vi "UHR-Fleezers Control (host) - 10.7.vi"() -> ()   [LabVIEW 2010] (continued)
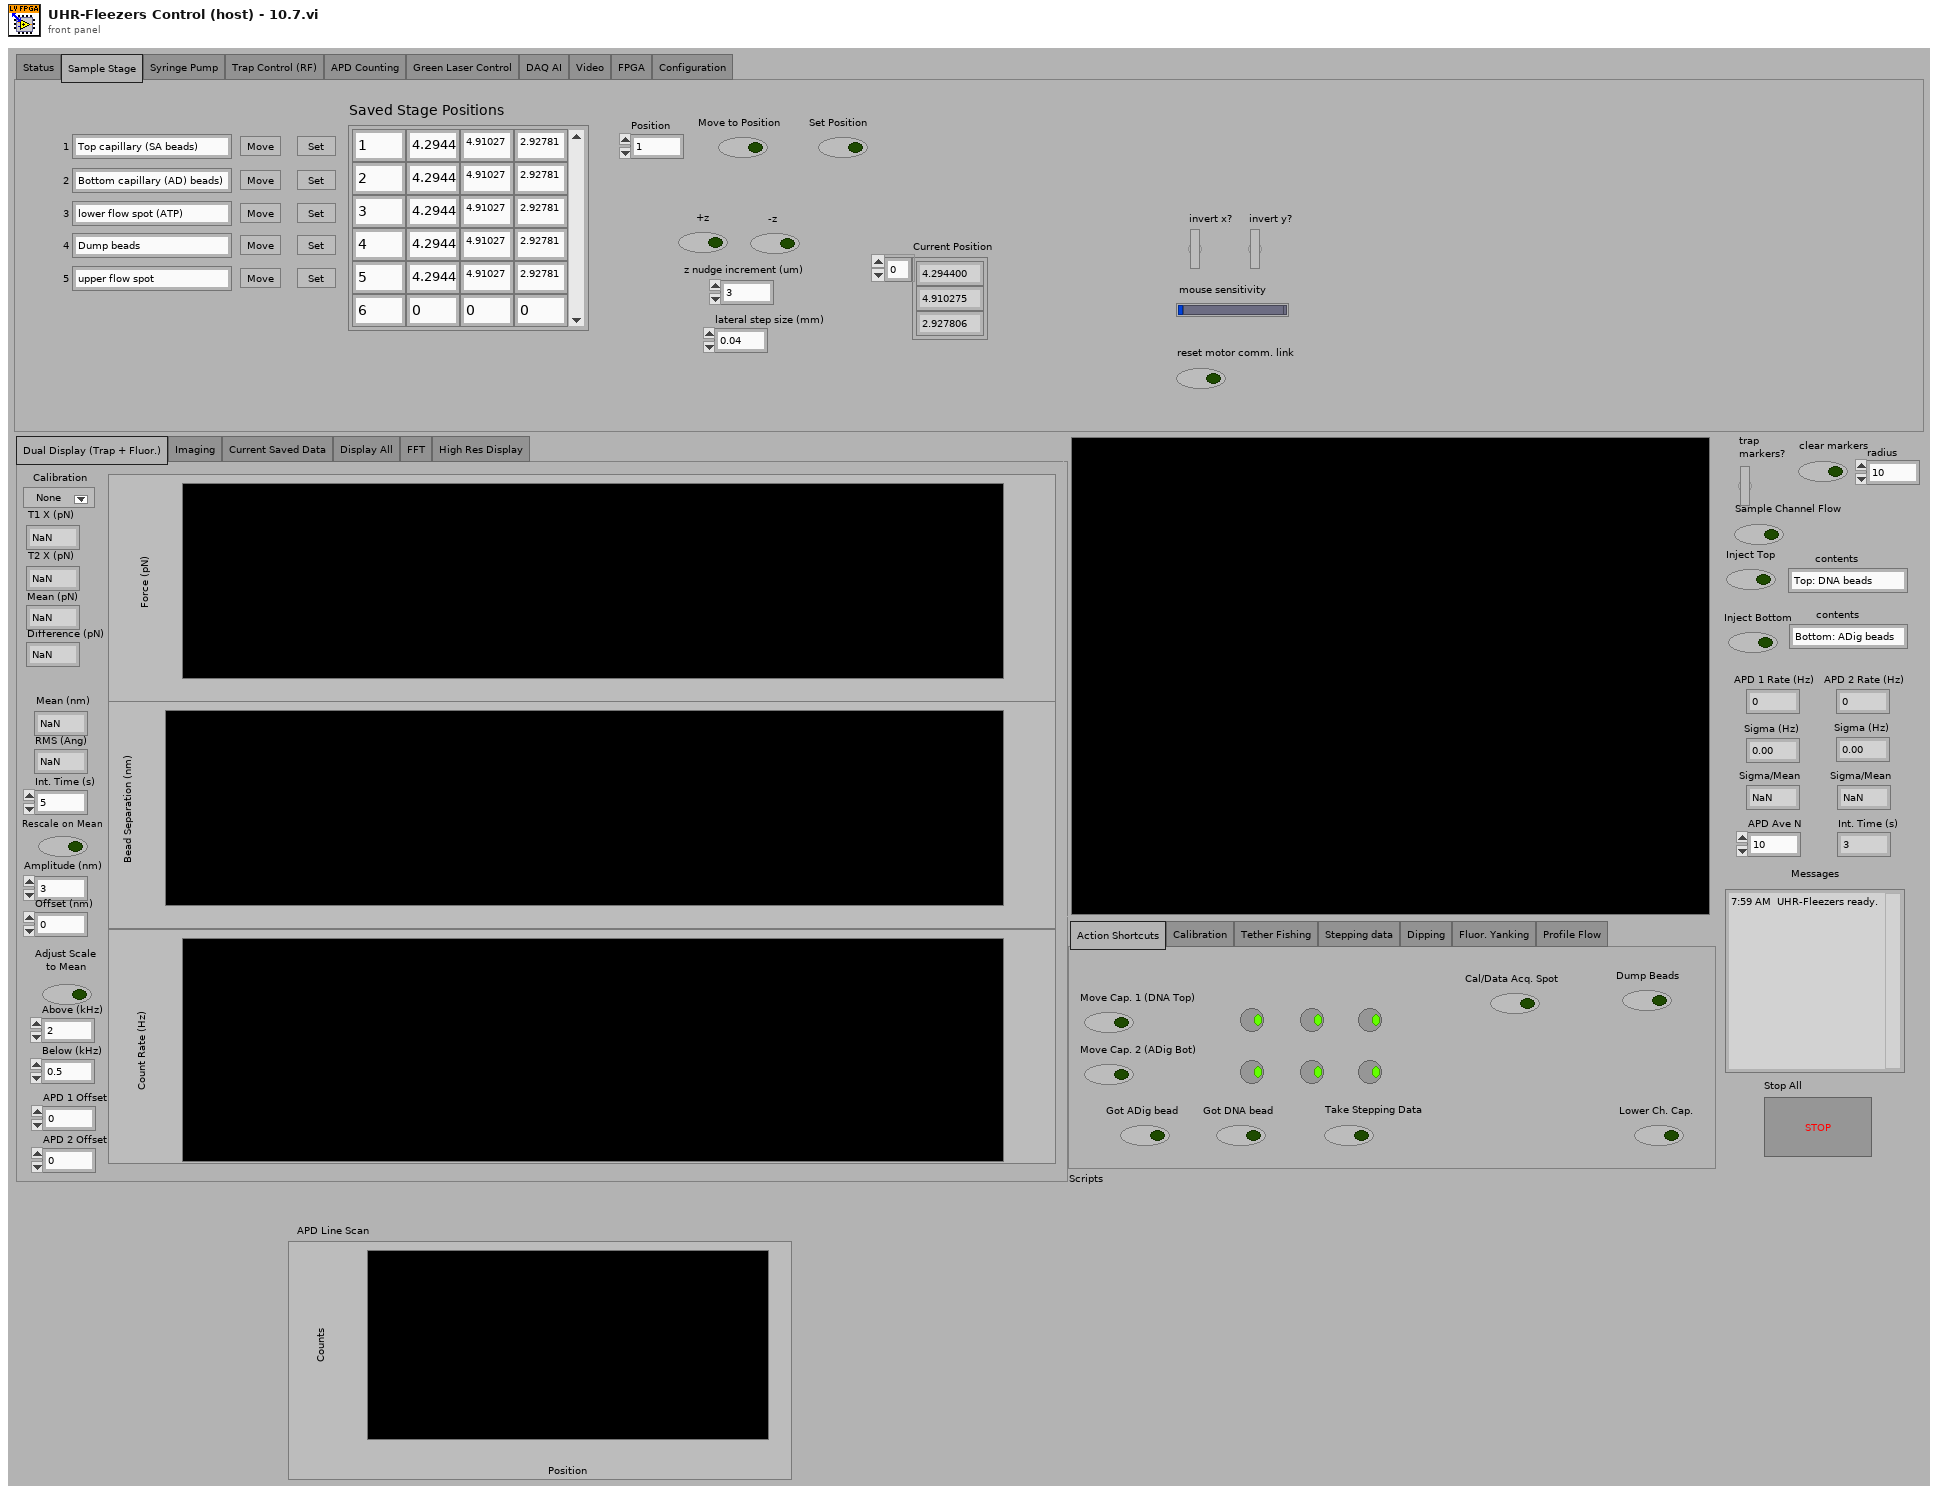
[diagram p1: front panel]
types:
  T1 = enum32{"Action Shortcuts", "Calibration", "Tether Fishing", "Stepping data", "Dipping", "Fluor. Yanking", "Profile Flow"}
  T2 = typedef "IMAQ Image.ctl" = refnum<image>
  T3 = enum32{"Dual Display (Trap + Fluor.)", "Imaging", "Current Saved Data", "Display All", "FFT", "High Res Display"}
  T4 = enum32{"Status", "Sample Stage", "Syringe Pump", "Trap Control (RF)", "APD Counting", "Green Laser Control", "DAQ AI", "Video", "FPGA", "Configuration"}
  T5 = cluster{"Pump 1":cluster{"Diameter (mm)":dbl, "Units":dbl, "Volume":dbl, "Rate":dbl}, "Pump 2":cluster{"Diameter (mm)":dbl, "Units":dbl, "Volume":dbl, "Rate":dbl}, "Pump 3":cluster{"Diameter (mm)":dbl, "Units":dbl, "Volume":dbl, "Rate":dbl}}
  T6 = enum32{"IR Laser Interlacing (Direct RF Board Control Method)", "AOD Raster Scan", "Feedback on Trap Intensity", "Feedback on Trap Position"}
  T7 = typedef "LVPoint32TypeDef.ctl" = cluster{"Horizontal":i32, "Vertical":i32}
  T8 = cluster{"Scan Range AOD (nm) 2":dbl, "Step Size AOD (nm) 2":dbl, "Scan Speed AOD (nm/s) 2":dbl, "Number of scans (AOD) 2":u16, "Label":string}[]
  T9 = cluster{"Set 1":cluster{"proportional gain (Kc)":i16, "integral gain (Kc*Ts/Ti)":i16, "derivative gain (Kc*Td/Ts)":i16}, "Set 2":cluster{"proportional gain (Kc)":i16, "integral gain (Kc*Ts/Ti)":i16, "derivative gain (Kc*Td/Ts)":i16}}
  T10 = cluster{"Trap 1":fxp<+/-,16,1>, "Trap 2":fxp<+/-,16,1>}
  T11 = cluster{"proportional gain (Kc)":fxp<+/-,16,8>, "integral gain (Kc*Ts/Ti)":fxp<+/-,16,8>, "derivative gain (Kc*Td/Ts)":fxp<+/-,16,8>}
  T12 = cluster{"output high":fxp<+/-,16,1>, "output low":fxp<+/-,16,1>}
  T13 = cluster{"Set 1":fxp<+/-,16,1>, "Set 2":fxp<+/-,16,1>}
  T14 = cluster{"proportional gain (Kc)":i16, "integral gain (Kc*Ts/Ti)":i16, "derivative gain (Kc*Td/Ts)":i16}
  T15 = cluster{"Set 1":bool, "Set 2":bool, "Set 3":bool}
  T16 = typedef "LVMinMaxIncTypeDef.ctl" = cluster{"Minimum":dbl, "Maximum":dbl, "Increment":dbl}
  T17 = typedef "Image Type" = u32
  T18 = typedef "nirio_resource_hc.ctl" = tag
  T19 = typedef "openfpgaref.8.6.ctl" = refnum<k20>
  T20 = typedef "niFpgaNodeNameForErrorReporting.ctl" = enum16{"Open FPGA VI Reference", "Read/Write Control", "Invoke Method: Abort", "Invoke Method: Acknowledge IRQ", "Invoke Method: Download", "Invoke Method: FIFO.Configure", "Invoke Method: FIFO.Read", "Invoke Method: FIFO.Start", "Invoke Method: FIFO.Stop", "Invoke Method: FIFO.Write", "Invoke Method: Reset", "Invoke Method: Run", "Invoke Method: Wait on IRQ", "Close FPGA VI Reference"}
  T21 = typedef "niLvFpgaWhatHappensToTopLevelVI.ctl" = enum16{"top level VI scripted behind XNode", "top level VI inlined behind XNode"}
  T22 = enum16{"GET STATUS", "ABS MOVE", "GET POS", "REL MOVE", "INIT", "CLOSE", "HOME", "READ ASCII", "ASCII", "SET ULIM", "STOP", "SET LLIM"}
  T23 = enum16{"CONNECT", "INITIALIZE VALVES", "DISCONNECT", "MOVE VALVE"}
  T24 = cluster{"New Image":T2, "New Image":T2, "New Image":T2, "New Image":T2}
  T25 = enum16{"open", "replace", "create", "open or create", "replace or create", "replace or create with confirmation"}
  T26 = typedef "XDNodeRunTimeDep.lvlib/timing_clust.ctl" = cluster{"Expected End [f-1]":u64, "Actual End [f-1]":u64, "Finished Late? [f-1]":bool, "Expected End [i-1]":u64, "Actual End [i-1]":u64, "Finished Late? [i-1]":bool, "Expected Start [i]":u64, "Actual Start [i]":u64, "Expected Start [f]":u64, "Actual Start [f]":u64, "Source Name":string, "Structure Name":string, "Period":i64, "Deadline":i64, "Offset":i64, "Start":i64, "Priority":i32, "Timeout":i32, "Mode":T27, "Wakeup Reason":T28, "Error":errorcluster, "Source Type":string, "Secondary Source Type":string, "Global End Time":u64, "Global Start Time":u64, "Frame Duration":u64, "Iteration Duration":u64, "Assigned CPU":i32, "I/O Scan Engine Mode":u32}
  T27 = typedef "XDNodeRunTimeDep.lvlib/nitl_modes.ctl" = enum32{"No Change", "Process missed periods, maintain original phase", "Discard missed periods, maintain original phase", "Process missed periods, ignore original phase", "Discard missed periods, ignore original phase"}
  T28 = typedef "XDNodeRunTimeDep.lvlib/wakeup.ctl" = enum32{"Normal", "Aborted", "Asynchronous wakeup", "Timing source error", "Timed loop error", "Timeout"}
  T29 = cluster{"[0]":i32, "[1]":i32, "[2]":i32, "[3]":i32}
  T30 = cluster{"[0]":i32, "[1]":i32, "[2]":i32, "[3]":i32}[]
  T31 = cluster{"Horizontal":i32, "Vertical":i32, "Scrolling":i32}
  T32 = enum32{"Normal Display", "Dual Display (APD)", "FFT", "High Res Display"}
  T33 = cluster{"Origin Pixel":cluster{"X":sgl, "Y":sgl}, "Angle Relative to Horizontal (deg)":sgl, "Axis Reference":u32}
  T34 = typedef "Simple Grid Descriptor" = cluster{"X Step":sgl, "Y Step":sgl, "Unit":T35}
  T35 = typedef "Image Unit" = enum32{"Undefined", "Angström", "Micrometer", "Millimeter", "Centimeter", "Meter", "Kilometer", "Microinch", "Inch", "Feet", "Nautical miles", "Standard miles", "Steps"}
  T36 = cluster{"averaging mode":u16, "weighting mode":u16, "number of averages":u32}
  T37 = cluster{"dB On (F)":bool, "unwrap phase (F)":bool, "convert to degree (F)":bool}
  T38 = cluster{"Green FB Ch 0":i16, "Green FB Ch 1":i16, "Green FB Ch 2":i16}
  T39 = enum16{"big-endian, network order", "native, host order", "little-endian"}
  T40 = cluster{string, string, string, string, string, string, string, string}
  T41 = cluster{string, string, string, string, string, string, string, string, string, string, string, string}
  T42 = cluster{string, string, string, string, string, string, string, string, string, string, string, string, string}
  T43 = cluster{string, string, string, string, string, string, string, string, string, string, string, string, string, string}
  T44 = cluster{"BD 1 Frequency 1 (MHz)":dbl, "BD 1 Frequency 2 (MHz)":dbl}
  T45 = cluster{"f0":dbl, "df":dbl, "magnitude":dbl[]}[][]
  T46 = cluster{"Green FB Ch 0":dbl, "Green FB Ch 1":dbl, "Green FB Ch 2":dbl}
  T47 = enum16{"Always On", "Always Off", "Off While Running"}
  T48 = cluster{"Scan Range AOD (nm) 2":dbl, "Step Size AOD (nm) 2":dbl, "Scan Speed AOD (nm/s) 2":dbl, "Number of scans (AOD) 2":u16, "Label":string}
  T49 = typedef "eventvkey.ctl" = enum16{"ASCII", "Enter", "Return", "Shift", "Ctrl", "Alt", "Cmd", "Opt", "Caps", "NumLock", "Clear", "Break", "Up", "Down", "Left", "Right", "Insert", "Delete", "Home", "End", "PageUp", "PageDown", "Escape", "Help", "Pause", "ScrollLock", "F1", "F2", "F3", "F4", "F5", "F6", "F7", "F8", "F9", "F10", "F11", "F12", "F13", "F14", "F15", "F16", "F17", "F18", "F19", "F20", "F21", "F22", "F23", "F24", "Play", "VolumeUp", "VolumeDown", "Mute", "Two Byte Char"}
  T50 = cluster{"[0]":dbl, "[1]":dbl, "[2]":dbl, "[3]":dbl, "[4]":dbl, "[5]":dbl}
  T51 = cluster{"Diameter (mm)":dbl, "Units":dbl, "Volume":dbl, "Rate":dbl}
  T52 = cluster{"Left":i32, "Top":i32, "Width":u32, "Height":u32}
  T53 = cluster{cluster{"Left":i32, "Top":i32, "Width":u32, "Height":u32}}[]
diagram:
  w63 = T17 2 items=["Grayscale (U8)", "Grayscale (I16)", "Grayscale (SGL)", "Complex (CSG)", "RGB (U32)", "HSL (U32)", "RGB (U64)", "Grayscale (U16)"] ("Image Type")
  w120 = cluster{"output high":i16, "output low":i16} {"output high"=3000, "output low"=0} ("FB output range 1")
  w195 = 10.0 ("y")
  w194 = 32767.0 ("y")
  w210 = 6.0  # clock mult.
  w211 = 49152000.0  # TCXO frequ.
  n1 = Build Array("DIO count 1 (ticks)", "DIO count 2 (ticks)", "DIO count 3 (ticks)") -> (w109:u32[])
  n2 = Multiply(x="APD Integration Time (s)", y=40000000.0) -> (x*y=w127:dbl)
  n3 = Reciprocal(x="APD Integration Time (s)") -> (1/x=w124:dbl)
  n4 = local write "APD Acq Rate (Hz)"(w124) -> ()
  n5 = local read "AO1"() -> (w189:dbl)
  n6 = local read "AO2"() -> (w188:dbl)
  n7 = To Unsigned Long Integer(number=w127) -> (unsigned 32bit integer=w126:u32)
  "APD Int. Count" <- w126
  n8 = local read "Scan Increment (MHz)"() -> (w206:dbl)
  n9 = local read "Continuous MCL Scanning"() -> (w176:bool)
  n10 = local read "Fast Scan Dir"() -> (w175:bool)
  n11 = local read "Trap Intensity\nSetpoints (V)"() -> (w225:cluster{"Set 1":dbl, "Set 2":dbl})
  n12 = local read "Number of scans (MCL)"() -> (w177:u64)
  n13 = Multiply(x=w189, y=w194) -> (x*y=w191:dbl)
  n14 = Multiply(x=w188, y=w194) -> (x*y=w193:dbl)
  n15 = Divide(x=w191, y=w195) -> (x/y=w190:dbl)
  n16 = Divide(x=w193, y=w195) -> (x/y=w192:dbl)
  n17 = To Word Integer(number=w190) -> (16bit integer=w187:i16)
  n18 = To Word Integer(number=w192) -> (16bit integer=w186:i16)
  n19 = Not(x=w175) -> (.not. x?=w170:bool)
  n20 = local read "Cycles/step (MCL)"() -> (w178:u64)
  n21 = Multiply(x=w206, y=1000.0) -> (x*y=w213:dbl)
  n22 = local read "Scan steps (MCL)"() -> (w179:u64)
  n23 = local write "Trap Pos FIFO Timeout"(u16 0 ("Trap Pos FIFO Timeout")) -> ()
  n24 = local read "Desired Scan Incr (V)"() -> (w181:dbl)
  n25 = Scale By Power Of 2(n=48, x=w213) -> (x*2^n=w214:dbl)
  n26 = Multiply(x=w211, y=w210) -> (x*y=w209:dbl)
  n27 = Divide(x=w214, y=w209) -> (x/y=w208:dbl)
  n28 = local read "Number Interlace Sets"() -> (w102:u8)
  n29 = Split 1D Array(array=w109, index=w102) -> (first subarray=w111:u32[])  [unwired: 1 out]
  n30 = Add Array Elements(numeric array=w111) -> (sum=w110:u32)
  n31 = property on="AI Count (ticks)" class="DigNum (strict)"("Val(Sgnl)"="AI Count (ticks)") -> ()  [unwired: 2 in, 2 out]
  n32 = local read "# Samples/channel"() -> (w198:u32)
  n33 = local read "Number of F/B Scans (AOD)"() -> (w199:u16)
  n34 = To Quad Integer(1:w208) -> (0:w205:i64)
  n35 = local read "Not-Interlacing Set"() -> (w101:enum32{"Set 1", "Set 2", "Set 3"})
  n36 = To Unsigned Byte Integer(number=w101) -> (unsigned 8bit integer=w107:u8)
  n37 = Index Array(array=w109, index=w107) -> (element=w108:u32)
  n38 = local read "Feedback On/Off"() -> (w228:cluster{"Set 1":bool, "Set 2":bool})
  n39 = local read "PID Gains"() -> (w220:T9)
  n40 = Divide(x=40000000.0, y="AI Count (ticks)") -> (x/y=w167:dbl)
  n41 = Multiply(x=w181, y=32767.0) -> (x*y=w183:dbl)
  n42 = local read "Scan steps (AOD)"() -> (w204:u64)
  n43 = local read "All FB On/Off"() -> (w229:bool)
  n44 = local read "Cycles/step (AOD)"() -> (w203:u64)
  n45 = local write "AI rate (Hz)"(w167) -> ()
  n46 = Divide(x=w183, y=10.0) -> (x/y=w182:dbl)
  n47 = Multiply(x=w204, y=w203) -> (x*y=w202:u64)
  n48 = Multiply(x=3276.7, y=w225) -> (x*y=w224:cluster{"Set 1":dbl, "Set 2":dbl})
  n49 = To Word Integer(number=w182) -> (16bit integer=w180:i16)
  n50 = Multiply(x=w202, y=u64 2) -> (x*y=w200:u64)
  n51 = local read "Sets to FIFO (Traps)"() -> (w232:T15)
  n52 = Divide(x=w167, y="FPGA Ave.") -> (x/y=w168:dbl)
  n53 = To Word Integer(number=w224) -> (16bit integer=w223:cluster{"Set 1":i16, "Set 2":i16})
  n54 = xnode "Open FPGA VI Reference"("resource name"=T18 "750kHzDAQ") -> ("FPGA VI Reference Out"=w217:T19)  [unwired: 1 in, 1 out]
  n55 = Unbundle By Name(w220) -> ("Set 1"=w219:T14, "Set 2"=w218:T14)
  n56 = Multiply(x=w200, y=w199) -> (x*y=w197:u64)
  n57 = local write "Ave. Rate (Hz)"(w168) -> ()
  n58 = Divide(x=w197, y=w198) -> (x/y=w196:dbl)
  n59 = Unbundle By Name(w223) -> ("Set 1"=w222:i16, "Set 2"=w221:i16)
  n60 = local read "2D or 1D Scan"() -> (w121:bool)
  n61 = local write "Data points/scans"(w197) -> ()
  n62 = local read "Scan BD"() -> (w215:bool)
  n63 = And(x=w228, y=w229) -> (x .and. y?=w227:cluster{"Set 1":bool, "Set 2":bool})
  n64 = local write "Data points/scan (f/b)"(w200) -> ()
  n65 = Reciprocal(x=w168) -> (1/x=w169:dbl)
  n66 = local read "N Acq Sets (Traps + Fl.)"() -> (w160:i16)
  n67 = local write "N sets should be saved"(w196) -> ()
  n68 = Unbundle By Name(w227) -> ("Set 1"=w231:bool, "Set 2"=w230:bool)
  n69 = local read "Interlace"() -> (w103:bool)
  n70 = Select(t=w110, s=w103, f=w108) -> (s? t:f=w100:u32)
  n71 = local write "Update Count (MCL)"(w100) -> ()
  n72 = local write "Total Counts (ticks)"(w100) -> ()
  n73 = xnode "Invoke Method"("FPGA VI Reference In"=w217) -> ("FPGA VI Reference Out"=w119:T19, "error out"=w138:errorcluster)  [unwired: 1 in]
  n74 = local write "Ave. Period (s)"(w169) -> ()
  n75 = property on="2D or 1D Scan" class="Bool (strict)"("Val(Sgnl)"=w121) -> ()  [unwired: 2 in, 2 out]
  n76 = xnode "Read/Write Control"("FPGA VI Reference In"=w118, "error in"=w138, "ai count"="AI Count (ticks)", "Interlace ON/OFF"=w103, "Number Interlace Cycles"=w102, "AI1 Sets to FIFO"=w232, "FB On/Off Set 1"=w231, "FB On/Off Set 2"=w230, "Interlace Off Parameters"=w101, "FB Setpoint Set 1"=w222, "FB Setpoint Set 2"=w221, "FB Gains Set 1"=w219, "FB Gains Set 2"=w218, "FB output range 1"=w120, "FB output range 2"=w120, "Cycles per step"=w203, "Scan BD"=w215, "Number of scans"=w199, "Scan steps"=w204, "Scan freq.  increment"=w205, "AO1"=w187, "AO2"=w186, "Scan freq.  increment (MCL)"=w180, "Scan steps (MCL)"=w179, "Cycles per step (MCL)"=w178, "Number of scans (MCL)"=w177, "MCL count"=w100, "Cont. Scan (MCL)"=w176, "MCL Scan Axis"=w170, "1D or 2D Scan?"=w121, "N of AI1 Int Acq Sets"=w160, "Freq or Amp switch first"="Freq or Amp switch first", "Freq switch delay"="Freq switch delay", "Amp switch delay"="Amp switch delay", "Swap F1 and F2"="Swap F1 and F2", "APD Acq Rate Count"=w126, "APD to FIFO"=FALSE, "APD Gate Operating Mode"="APD Gate", "APD Gate ON Count"="APD Gate ON Count", "APD Gate OFF Count"="APD Gate OFF Count", "Invert APD Gate"="Invert APD Gate", "DIO count 1 (ticks)"="DIO count 1 (ticks)", "DIO count 2 (ticks)"="DIO count 2 (ticks)", "DIO count 3 (ticks)"="DIO count 3 (ticks)", "APD 1 AO scale factor"="APD 1 AO Mult.", "APD 2 AO scale factor"="APD 2 AO Mult.") -> ("FPGA VI Reference Out"=w95:T19, "error out"=w97:errorcluster)  [unwired: 1 in]
  n77 = local read "Green Laser ON/Interlacing"() -> (w98:bool)
  n78 = local read "Green laser mode"() -> (w99:enum32{"Laser ON", "Laser OFF", "Interlace"})
  n79 = local read "GI Frequency, OFF count"() -> (w91:u32)
  n80 = local read "GI Frequency, ON count"() -> (w90:u32)
  n81 = Multiply(x="Current When FB OFF (%)", y=655.35) -> (x*y=w81:dbl)
  n82 = local read "Green FB Count"() -> (w89:u32)
  n83 = Multiply(x="Green FB Setpoint (mV)", y=3.2767) -> (x*y=w78:dbl)
  n84 = To Unsigned Word Integer(number=w81) -> (unsigned 16bit integer=w79:u16)
  n85 = local read "Invert GI"() -> (w93:bool)
  n86 = To Word Integer(number=w78) -> (16bit integer=w76:i16)
  n87 = case shown="True" w98 {
    tunnel: w99 -> [_ w252]
    tunnel: [enum32{"Laser ON", "Laser OFF", "Interlace"}."Laser OFF" ("Green laser mode") w252] -> w92
    frame False {
    }
    frame True {
    }
  }
  n88 = local read "Trap Pos. AI1 X Pre-scale"() -> (w47:u16)
  n89 = local read "Trap Pos FB Monitor\nT1 or T2"() -> (w54:bool)
  n90 = local read "Trap Pos FB Int Count"() -> (w42:u16)
  n91 = local read "Trap Pos FB Negate Action"() -> (w53:bool)
  n92 = local read "Trap Pos. FB Offset Factor"() -> (w52:i64)
  n93 = local read "Trap Pos. FB Mult Factor"() -> (w51:i64)
  n94 = local read "Trap Pos. FB Gains"() -> (w49:T11)
  n95 = local read "Trap Pos. FB Range"() -> (w50:T12)
  n96 = xnode "Read/Write Control"("FPGA VI Reference In"=w95, "error in"=w97, "Green interlace ON count 2"=w90, "Green interlace OFF count 2"=w91, "Invert GI 2"=w93, "Operating Mode 2"=w92, "Green FB Gains"="Green FB Gains", "Green FB Setpoint"=w76, "Green FB On/Off"="Green FB On/Off", "Current Out"=w79, "Green int current ON count adj"="Green int current ON count adj", "Green FB Count"=w89, "Operating Mode"=w92, "Green interlace OFF count"=w91, "Green interlace ON count"=w90, "Invert GI"=w93, "Trap Pos FB Monitor T1 or T2"=w54, "Trap Pos FB Negate Action"=w53, "Trap Pos. FB Offset Factor"=w52, "Trap Pos. FB Mult Factor"=w51, "Trap Pos. FB Range"=w50, "Trap Pos. FB Gains"=w49, "Force feedback"=FALSE, "AI1 X Scale"=w47, "Trap Pos to FIFO"=TRUE, "Trap Pos FB Int Count"=w42) -> ("FPGA VI Reference Out"=w94:T19, "error out"=w96:errorcluster)
  n97 = xnode "Invoke Method"("FPGA VI Reference In"=w94, "error in"=w96, "Depth"="Trap AI FIFO Depth") -> ("FPGA VI Reference Out"=w57:T19, "error out"=w56:errorcluster)
  n98 = xnode "Invoke Method"("FPGA VI Reference In"=w57, "error in"=w56, "Depth"="Trap Position FIFO Depth") -> ("FPGA VI Reference Out"=w44:T19, "error out"=w43:errorcluster)
  n99 = flat-sequence {
    tunnel: w119 -> [w257]
    tunnel: [w257] -> w118
    tunnel: [w256] -> w117
    tunnel: [w255] -> w116
    tunnel: [w253] -> w114
    tunnel: [w254] -> w115
    frame #0 {
      w254 = T16 {"Minimum"=50.0, "Maximum"=100.0, "Increment"=1.0} ("Min Max Inc")
      w253 = T16 {"Minimum"=0.0, "Maximum"=75.0, "Increment"=1.0} ("Data Entry Limits")
      w256 = T16 {"Minimum"=50.0, "Maximum"=100.0, "Increment"=1.0} ("Min Max Inc")
      w255 = T16 {"Minimum"=0.0, "Maximum"=75.0, "Increment"=1.0} ("Data Entry Limits")
      n100 = property on="BD 2 Frequency 1 (MHz)" class="DigNum (strict)"("Data Range"=w254) -> ()  [unwired: 2 in, 2 out]
      n101 = property on="BD 2 Frequency 3 (MHz)" class="DigNum (strict)"("Data Range"=w254) -> ()  [unwired: 2 in, 2 out]
      n102 = property on="BD 2 Frequency 2 (MHz)" class="DigNum (strict)"("Data Range"=w254) -> ()  [unwired: 2 in, 2 out]
      n103 = property on="BD 1 Frequency 1 (MHz)" class="DigNum (strict)"("Data Range"=w256) -> ()  [unwired: 2 in, 2 out]
      n104 = property on="BD 1 Frequency 2 (MHz)" class="DigNum (strict)"("Data Range"=w256) -> ()  [unwired: 2 in, 2 out]
      n105 = property on="BD 1 Frequency 3 (MHz)" class="DigNum (strict)"("Data Range"=w256) -> ()  [unwired: 2 in, 2 out]
      n106 = property on="BD 2 Amplitude 1 (%)" class="DigNum (strict)"("Data Range"=w253) -> ()  [unwired: 2 in, 2 out]
      n107 = property on="BD 2 Amplitude 2 (%)" class="DigNum (strict)"("Data Range"=w253) -> ()  [unwired: 2 in, 2 out]
      n108 = property on="BD 2 Amplitude 3 (%)" class="DigNum (strict)"("Data Range"=w253) -> ()  [unwired: 2 in, 2 out]
      n109 = property on="BD 1 Amplitude 3 (%)" class="DigNum (strict)"("Data Range"=w255) -> ()  [unwired: 2 in, 2 out]
      n110 = property on="BD 1 Amplitude 2 (%)" class="DigNum (strict)"("Data Range"=w255) -> ()  [unwired: 2 in, 2 out]
      n111 = property on="BD 1 Amplitude 1 (%)" class="DigNum (strict)"("Data Range"=w255) -> ()  [unwired: 2 in, 2 out]
      "X RF Frequency Limits (MHz)" <- w256
      "X RF Amplitude Limits (%)" <- w255
      "Y RF Amplitude Limits (%)" <- w253
      "Y RF Frequency Limits (MHz)" <- w254
    }
  }
  n112 = xnode "Invoke Method"("FPGA VI Reference In"=w44, "error in"=w43) -> ("FPGA VI Reference Out"=w14:T19, "error out"=w13:errorcluster)  [unwired: 1 out]
  n113 = flat-sequence "Initial FPGA Loop Relative Phase Adjustment" {
    tunnel: "Initial Phase Adjustment (APD 2 Gate)" -> [w259]
    tunnel: "Initial Phase Adjustment (GI) 2" -> [w260]
    tunnel: "Initial Phase Adj. (MCL)" -> [w261]
    tunnel: w13 -> [w262]
    tunnel: w14 -> [w263]
    tunnel: "Initial Phase Adjustment (GI)" -> [w264]
    tunnel: "Initial Phase Adjustment (AI1)" -> [w265]
    tunnel: [w265] -> w28
    tunnel: [w264] -> w27
    tunnel: [w263] -> w26
    tunnel: [w262] -> w25
    tunnel: [w261] -> w24
    tunnel: [w260] -> w23
    tunnel: [w259] -> w22
    tunnel: [w277] -> w144
    tunnel: [w271] -> w142
    tunnel: "Initial Phase Adjustment (APD Acq)" -> [w270]
    tunnel: "Initial Phase Adjustment (APD 1 Gate)" -> [w269]
    tunnel: "Initial Phase Adjustment (Green FB)" -> [w268]
    tunnel: w28 -> [w276]
    tunnel: w27 -> [w275]
    tunnel: w26 -> [w274]
    tunnel: w25 -> [w273]
    tunnel: w24 -> [w272]
    tunnel: w23 -> [w267]
    tunnel: w22 -> [w266]
    tunnel: w144 -> [w456]
    tunnel: [w457] -> w143
    tunnel: w142 -> [w457]
    tunnel: [w456] -> w141
    tunnel: w143 -> [w460]
    tunnel: w141 -> [w459]
    tunnel: [w462] -> w140
    tunnel: [w461] -> w139
    tunnel: [w649] -> w12
    tunnel: [w650] -> w15
    tunnel: w140 -> [w650]
    tunnel: w139 -> [w649]
    frame #0 {
      n114 = Wait (ms)(milliseconds to wait=u32 1000) -> ()  [unwired: 1 out]
    }
    frame #1 {
      n115 = xnode "Read/Write Control"("FPGA VI Reference In"=w274, "error in"=w273, "Phase count adjustment"=w276, "Phase count adjustment (GI)"=w275, "Phase count adjustment (MCL)"=w272, "Phase Count Adjustment (APD Acq)"=w270, "Phase count adjustment (APD 1 Gate)"=w269, "Phase count adjustment (APD 2 Gate)"=w266, "Phase count adjustment (Green FB)"=w268, "Phase count adjustment (GI) 2"=w267) -> ("FPGA VI Reference Out"=w271:T19, "error out"=w277:errorcluster)
    }
    frame #2 {
      n116 = Wait (ms)(milliseconds to wait=u32 1000) -> ()  [unwired: 1 out]
    }
    frame #3 {
      w458 = TRUE
      n117 = xnode "Read/Write Control"("FPGA VI Reference In"=w460, "error in"=w459, "+ phase"=w458, "+ phase (GI)"=w458, "+ phase (MCL)"=w458, "+ phase (APD Acq)"=w458, "+ phase (APD 1 Gate)"=w458, "+ phase (APD 2 Gate)"=w458, "+ phase (Green FB)"=w458, "+ phase (GI) 2"=w458) -> ("FPGA VI Reference Out"=w461:T19, "error out"=w462:errorcluster)
    }
    frame #4 {
      n118 = Wait (ms)(milliseconds to wait=u32 1000) -> ()  [unwired: 1 out]
    }
  }
  n119 = local read "Phase adj. (Green FB)"() -> (w112:i16)
  n120 = local read "Phase adj. (GI) 2"() -> (w82:i16)
  n121 = local read "Phase adjust (MCL)"() -> (w171:i16)
  n122 = local read "Phase adj. (AI1)"() -> (w173:i16)
  n123 = local read "Phase adj. (GI)"() -> (w172:i16)
  n124 = xnode "Read/Write Control"("FPGA VI Reference In"=w12, "error in"=w15, "Phase count adjustment"=w173, "Phase count adjustment (GI)"=w172, "Phase count adjustment (MCL)"=w171, "Phase Count Adjustment (APD Acq)"="Phase Adj. (APD Acq)", "Phase count adjustment (APD 1 Gate)"="Phase Adj. (APD 1 Gate)", "Phase count adjustment (APD 2 Gate)"="Phase Adj. (APD 2 Gate)", "Phase count adjustment (Green FB)"=w112, "Phase count adjustment (GI) 2"=w82) -> ("FPGA VI Reference Out"=w11:T19, "error out"=w10:errorcluster)
  n125 = call "Initialize RF boards - interlace 3.vi"("error in"=w10, "FPGA VI Reference In"=w11) -> ("FPGA VI Reference Out"=w149:T19)  [unwired: 1 out]
  n126 = call "set RF board frequency - interlace.vi"("Board 2 Frequency Limits"=w115, "Board 1 Frequency Limits"=w117, "FPGA VI Reference In"=w149, "Board 2 Frequency 3 (MHz)"="BD 2 Frequency 3 (MHz)", "Board 1 Frequency 3 (MHz)"="BD 1 Frequency 3 (MHz)", "Board 2 Frequency 2 (MHz)"="BD 2 Frequency 2 (MHz)", "Board 2 Frequency 1 (MHz)"="BD 2 Frequency 1 (MHz)", "Board 1 Frequency 2 (MHz)"="BD 1 Frequency 2 (MHz)", "Board 1 Frequency 1  (MHz)"="BD 1 Frequency 1 (MHz)") -> ("error out"=w243:errorcluster, "FPGA VI Reference Out"=w244:T19)  [unwired: 1 in]
  n127 = call "set RF board amplitude - interlace.vi"("Board 2 Amplitude Limits"=w114, "Board 1 Amplitude Limits"=w116, "error in"=w243, "FPGA VI Reference In"=w244, "Board 2 Amplitude 3 (%)"="BD 2 Amplitude 3 (%)", "Board 1 Amplitude 3 (%)"="BD 1 Amplitude 3 (%)", "Board 2 Amplitude 2 (%)"="BD 2 Amplitude 2 (%)", "Board 2 Amplitude 1 (%)"="BD 2 Amplitude 1 (%)", "Board 1 Amplitude 2 (%)"="BD 1 Amplitude 2 (%)", "Board 1 Amplitude 1 (%)"="BD 1 Amplitude 1 (%)") -> ("error out"=w8:errorcluster, "FPGA VI Reference Out"=w9:T19)
  n128 = flat-sequence {
    tunnel: w9 -> [w659]
    tunnel: w8 -> [w658]
    tunnel: [w657] -> w236
    tunnel: [w656] -> w235
    tunnel: [w701] -> w234
    tunnel: w236 -> [w701]
    tunnel: [w700] -> w233
    tunnel: w235 -> [w700]
    tunnel: w234 -> [w710]
    tunnel: w233 -> [w709]
    tunnel: [w708] -> w38
    tunnel: [w707] -> w37
    tunnel: w38 -> [w775]
    tunnel: w37 -> [w770]
    tunnel: [w775] -> w2
    tunnel: [w750] -> w1
    tunnel: [w776] -> w39
    tunnel: [w781] -> w16
    tunnel: w2 -> [w781]
    tunnel: w1 -> [w778]
    frame #0 {
      n129 = local read "Trap 1 (ON/OFF)"() -> (w651:bool)
      n130 = xnode "Read/Write Control"("FPGA VI Reference In"=w659, "error in"=w658, "Direct RF Box  Communication"=FALSE) -> ("FPGA VI Reference Out"=w657:T19, "error out"=w656:errorcluster)
      n131 = local write "Saving..."(FALSE ("Saving Data")) -> ()
      n132 = local write "Stop All"(FALSE ("Stop All")) -> ()
      n133 = local write "Index"(1.0 ("Index")) -> ()
      n134 = property on="Trap 1 ON" class="Bool (strict)"("Value"=w651) -> ()  [unwired: 2 in, 2 out]
      "Manipulating Trap" <- FALSE ("Manipulating Trap")
    }
    frame #1 {
      n135 = local read "Trap 2 (ON/OFF)"() -> (w699:bool)
      n136 = Wait (ms)(milliseconds to wait=u32 50) -> ()  [unwired: 1 out]
      n137 = property on="Trap 2 ON" class="Bool (strict)"("Val(Sgnl)"=w699) -> ()  [unwired: 2 in, 2 out]
    }
    frame #2 {
      n138 = local read "Scan Range (nm)"() -> (w703:dbl)
      n139 = xnode "Read/Write Control"("FPGA VI Reference In"=w710, "error in"=w709, "FPGA Controls  RF Box"=TRUE ("Direct RF Box  Communication")) -> ("FPGA VI Reference Out"=w708:T19, "error out"=w707:errorcluster)
      n140 = call "Update messages.vi"("Message to add"="UHR-Fleezers ready.", "Old message string"="") -> ("New message string"=w706:string)
      n141 = local write "Messages"(w706) -> ()
      n142 = property on="Scan Range (nm)" class="DigNum (strict)"("Val(Sgnl)"=w703) -> ()  [unwired: 2 in, 2 out]
    }
    frame #3 {
      w756 = T22."ASCII" ("Command")
      # "disable hysteresis\ncompensation for\nfaster performance"
      # "increase jerk\nfor faster \nresponse"
      # "disable backlash\ncompensation for\nfaster response \ntimes. necessary\nfor mouse control\nof stage"
      n143 = call "CONEX_FUNCTIONAL_GLOBAL.vi"("error in"=w770, "Command"=T22."INIT") -> ("error out"=w752:errorcluster)  [unwired: 7 in, 2 out]
      n144 = call "CONEX_FUNCTIONAL_GLOBAL.vi"("error in"=w752, "Position"=dbl[] [10.0, 12.0, 2.0], "Command"=T22."SET ULIM") -> ("error out"=w771:errorcluster)  [unwired: 6 in, 2 out]
      n145 = call "CONEX_FUNCTIONAL_GLOBAL.vi"("error in"=w771, "Position"=dbl[] [0.0, 0.0, 4.0], "Command"=T22."SET LLIM") -> ("error out"=w765:errorcluster)  [unwired: 6 in, 2 out]
      n146 = Concatenate Strings("1BA0", "\r\n") -> (w762:string)
      n147 = call "CONEX_FUNCTIONAL_GLOBAL.vi"("error in"=w765, "ASCII command"=w762, "Command"=w756) -> ("error out"=w761:errorcluster)  [unwired: 6 in, 2 out]
      n148 = Concatenate Strings("1JR0.001", "\r\n") -> (w758:string)
      n149 = call "CONEX_FUNCTIONAL_GLOBAL.vi"("error in"=w761, "ASCII command"=w758, "Command"=w756) -> ("error out"=w757:errorcluster)  [unwired: 6 in, 2 out]
      n150 = Concatenate Strings("1BH0", "\r\n") -> (w753:string)
      n151 = call "CONEX_FUNCTIONAL_GLOBAL.vi"("error in"=w757, "ASCII command"=w753, "Command"=w756) -> ("error out"=w751:errorcluster)  [unwired: 6 in, 2 out]
      n152 = call "CONEX_FUNCTIONAL_GLOBAL.vi"("error in"=w751, "Command"=T22."GET POS") -> ("error out"=w750:errorcluster, "Current Position"=w766:dbl[])  [unwired: 7 in, 1 out]
      n153 = local write "Current Position"(w766) -> ()
    }
    frame #4 {
      n154 = call "hamilton_controller.vi"("error in"=w778, "action"=T23."CONNECT") -> ("error out"=w777:errorcluster)  [unwired: 9 in]
      n155 = call "hamilton_controller.vi"("error in"=w777, "action"=T23."INITIALIZE VALVES") -> ("error out"=w776:errorcluster)  [unwired: 9 in]
    }
  }
  n156 = Subtract(x="BD 1 Frequency 1 (MHz)", y="BD 1 Frequency 2 (MHz)") -> (x-y=w159:dbl)
  n157 = Subtract(x="BD 2 Frequency 1 (MHz)", y="BD 2 Frequency 2 (MHz)") -> (x-y=w158:dbl)
  n158 = Square(x=w158) -> (x^2=w156:dbl)
  n159 = Square(x=w159) -> (x^2=w157:dbl)
  n160 = Add(x=w157, y=w156) -> (x+y=w155:dbl)
  n161 = Square Root(x=w155) -> (sqrt(x)=w154:dbl)
  n162 = local write "Trap Delta (MHz)"(w154) -> ()
  n163 = call "IMAQ Create"("Image Name"="APD 1 Image", "Image Type"=w63) -> ("New Image"=w62:T2)  [unwired: 3 in, 1 out]
  n164 = call "IMAQ Create"("Image Name"="APD 2 Image", "Image Type"=w63) -> ("New Image"=w61:T2)  [unwired: 3 in, 1 out]
  n165 = call "IMAQ Create"("Image Name"="Det. X Image", "Image Type"=w63) -> ("New Image"=w60:T2)  [unwired: 3 in, 1 out]
  n166 = call "IMAQ Create"("Image Name"="Det. Y Image", "Image Type"=w63) -> ("New Image"=w59:T2)  [unwired: 3 in, 1 out]
  n167 = Bundle("New Image"=w62, "New Image"=w61, "New Image"=w60, "New Image"=w59) -> (w58:T24)  [unwired: 1 in]
  n168 = disable-structure shown="Disabled" {
    disable-tunnel: w16 -> [w810 _]
    frame Disabled {
      w805 = T17 0 items=["Grayscale (U8)", "Grayscale (I16)", "Grayscale (SGL)", "Complex (CSG)", "RGB (U32)", "HSL (U32)", "RGB (U64)", "Grayscale (U16)"] ("Image Type")
      n169 = call <vilib>:"IMAQ Init.vi"("Interface Name"="img0") -> ("error out"=w807:errorcluster, "IMAQ Session Out"=w809:refnum<k11>)  [unwired: 9 in]
      n170 = call <vilib>:"IMAQ Grab Setup.vi"("error in (no error)"=w807, "IMAQ Session In"=w809) -> ("error out"=w803:errorcluster, "IMAQ Session Out"=w804:refnum<k11>)  [unwired: 8 in]
      n171 = call "IMAQ Create"("Image Name"="untitled", "Image Type"=w805) -> ("New Image"=w802:T2)  [unwired: 3 in, 1 out]
      n172 = call <vilib>:"Application Directory.vi"() -> ("Application Directory"=w789:path)
      n173 = Build Path(base path=w789, name or relative path="_trap_screen_positions") -> (appended path=w797:path)
      n174 = Open/Create/Replace File(file path (use dialog)=w797, operation (0:open)=T25."open or create", access (0:read/write)=enum16{"read/write", "read-only", "write-only"}."read/write") -> (refnum out=w799:refnum<file>)  [unwired: 3 in, 2 out]
      n175 = local read "Trap Sets"() -> (w791:u32)
      n176 = for "Load trap positions on video screen from file." {
        N: w791 -> [_]
        tunnel: [w817] -> w792
        tunnel: w799 -> [w816]
        tunnel: [w813] -> w788 mode=indexing
        w815 = 4
        n177 = for {
          N: w815 -> [_]
          tunnel: [w821] -> w817
          tunnel: w816 -> [w820]
          tunnel: w815 -> [w819]
          tunnel: [w818] -> w814 mode=indexing
          n178 = Read from Binary File(5:w819, 11:w820) -> (2:w818:i32, 3:w821:refnum<file>)  [unwired: 4 in, 2 out]
        }
        n179 = Array To Cluster(array=w814) -> (cluster=w813:T29)
      }
      n180 = node-c288() -> (w812:T26)  [unwired: 4 in]
      n181 = timed-loop "acquire video and stage position" {
        timing: w812 -> [_]
        timing-out: [_] -> w811
        tunnel: w804 -> [w840]
        tunnel: w803 -> [w839]
        tunnel: w802 -> [w838]
        tunnel: [w837] -> w784
        tunnel: [w834] -> w785
        tunnel: [w835] -> w783
        tunnel: w810 -> [_]
        shift-right: [w831] -> w801
        shift-left: w788 -> [w832]
        tunnel: w791 -> [w829]
        stop <- w836 stop-if-true
        n182 = node-c288() -> ()  [unwired: 1 in, 1 out]
        n183 = event shown="[2] \"Primary Video Display\": Mouse Down" {
          selector: _ -> [_ _ _ _]
          dyn-events: _ -> [_ _ _ _]
          timeout: 10 -> [_ _ _ _]
          tunnel: w840 -> [w851 w866 w875 w894]
          tunnel: w839 -> [w850 w868 w873 w896]
          tunnel: w838 -> [w849 w867 w874 w895]
          tunnel: [w848 w866 w875 w894] -> w837
          tunnel: [w841 w870 FALSE FALSE] -> w836
          tunnel: [w845 w868 w873 w896] -> w835
          tunnel: [w844 w867 w874 w895] -> w834
          tunnel: "radius" -> [_ _ w880 _]
          tunnel: w832 -> [w842 w869 w878 _]
          tunnel: [w842 w869 w879 cluster{i32, i32, i32, i32}[] []] -> w831
          tunnel: w829 -> [_ _ w871 _]
          event Timeout {
            n184 = event-data() -> ()  [unwired: 1 in, 2 out]
            n185 = call <vilib>:"IMAQ Grab Acquire.vi"("error in (no error)"=w850, "Image In"=w849, "IMAQ Session In"=w851) -> ("error out"=w846:errorcluster, "Image Out"=w847:T2, "IMAQ Session Out"=w848:refnum<k11>)  [unwired: 5 in, 1 out]
            n186 = case shown="True" "trap\nmarkers?" {
              tunnel: w842 -> [_ w859]
              tunnel: w847 -> [w853 w858]
              tunnel: w846 -> [w852 w857]
              tunnel: [w852 w856] -> w845
              tunnel: [w853 w854] -> w844
              frame False {
              }
              frame True {
                n187 = for {
                  tunnel: w859 -> [w865] mode=indexing
                  shift-right: [w863] -> w854
                  shift-left: w858 -> [w864]
                  tunnel: w857 -> [w862]
                  tunnel: [w861] -> w856
                  tunnel: u32 16711680 ("Color") -> [w860]
                  n188 = call "IMAQ Overlay Oval"("Color"=w860, "error in (no error)"=w862, "Bounding Rectangle"=w865, "Image"=w864) -> ("error out"=w861:errorcluster, "Image Out"=w863:T2)  [unwired: 6 in]
                }
              }
            }
            "Primary Video Display" <- w844
            n189 = Unbundle By Name(w846) -> ("status"=w841:bool)
          }
          event "Stop All": Value Change {
            n190 = event-data() -> ()  [unwired: 1 in, 5 out]
            n191 = local read "Stop All"() -> (w870:bool)
          }
          event "Primary Video Display": Mouse Down {
            n192 = event-data() -> ()  [unwired: 1 in, 7 out]
            n193 = Array Size(array=w878) -> (size(s)=w877:i32)
            n194 = Less?(x=w877, y=w871) -> (x < y?=w876:bool)
            n195 = case shown="True" w876 {
              tunnel: w880 -> [_ w890]
              tunnel: w878 -> [w881 w884]
              tunnel: [w881 w883] -> w879
              frame False {
              }
              frame True {
                n196 = property on="Primary Video Display" class="ImageControl"() -> ("Last Mouse Position"=w882:cluster{"X":i32, "Y":i32})  [unwired: 2 in, 2 out]
                n197 = Unbundle By Name(w882) -> ("X"=w892:i32, "Y"=w891:i32)
                n198 = Add(x=w891, y=w890) -> (x+y=w888:i32)
                n199 = Subtract(x=w891, y=w890) -> (x-y=w886:i32)
                n200 = Add(x=w892, y=w890) -> (x+y=w887:i32)
                n201 = Subtract(x=w892, y=w890) -> (x-y=w889:i32)
                n202 = Bundle(w889, w888, w887, w886) -> (w885:cluster{i32, i32, i32, i32})  [unwired: 1 in]
                n203 = Build Array (concatenate)(w884, w885) -> (w883:T30)
              }
            }
          }
          event "clear markers": Value Change {
            n204 = event-data() -> ()  [unwired: 1 in, 5 out]
          }
        }
        n205 = node-c288() -> ()  [unwired: 1 in, 1 out]
      }
      n206 = node-c288(w811) -> ()  [unwired: 1 out]
      n207 = Set File Position(offset (in bytes) (0)=i64 0, refnum=w792, from (0:start)=enum16{"start", "end", "current"}."start") -> (refnum out=w793:refnum<file>)  [unwired: 1 in, 1 out]
      n208 = for "Write trap positions to file so they can be remembered\nwhen program is removed from memory" {
        tunnel: w801 -> [w825] mode=indexing
        tunnel: [w823] -> w800
        tunnel: w793 -> [w822]
        n209 = Cluster To Array(cluster=w825) -> (array=w824:i32[])
        n210 = for {
          tunnel: w824 -> [w828] mode=indexing
          tunnel: [w827] -> w823
          tunnel: w822 -> [w826]
          n211 = Write to Binary File(file (use dialog)=w826, data=w828) -> (refnum out=w827:refnum<file>)  [unwired: 4 in, 2 out]
        }
      }
      n212 = Close File(refnum=w800) -> ()  [unwired: 1 in, 2 out]
      n213 = call "IMAQ Dispose"("Image"=w785, "error in (no error)"=w783) -> ("error out"=w782:errorcluster)  [unwired: 4 in]
      n214 = call <vilib>:"IMAQ Stop.vi"("error in (no error)"=w782, "IMAQ Session In"=w784) -> ("error out"=w786:errorcluster, "IMAQ Session Out"=w787:refnum<k11>)  [unwired: 8 in]
      n215 = call <vilib>:"IMAQ Close.vi"("error in (no error)"=w786, "IMAQ Session In"=w787) -> ()  [unwired: 9 in, 1 out]
    }
    frame Enabled {
    }
  }
  n216 = call <vilib>:"Initialize Mouse.vi"() -> ("error out"=w18:errorcluster, "device ID"=w19:refnum<k1>)  [unwired: 10 in]
  n217 = node-c288() -> (w4:T26)  [unwired: 4 in]
  n218 = call-poly <vilib>:"Acquire Input Data.vi"("device ID"=w19, "error in (no error)"=w18) -> ("device ID"=w20:refnum<k1>, "error out"=w17:errorcluster)  [unwired: 14 in, 2 out]
  n219 = timed-loop {
    tunnel: w20 -> [w909]
    tunnel: [w908] -> w21
    tunnel: [w907] -> _
    tunnel: w17 -> [w906]
    tunnel: w16 -> [_]
    shift-right: ["Use mouse to move stage\n(press mouse wheel to quit)"] -> _
    shift-left: _ -> [w903]
    timing: w4 -> [_]
    timing-out: [_] -> w3
    i -> [w902]
    stop <- w905 stop-if-true
    n220 = node-c288() -> ()  [unwired: 1 in, 1 out]
    n221 = case shown="True" "Use mouse to move stage\n(press mouse wheel to quit)" {
      tunnel: w909 -> [w919 w937]
      tunnel: [w919 w960] -> w908
      tunnel: [w912 w941] -> w907
      tunnel: w906 -> [w913 w935]
      tunnel: w903 -> [_ w938]
      tunnel: w902 -> [_ w933]
      frame False {
        n222 = case shown="True" "reset motor comm. link" {
          tunnel: [w920 w923] -> w914
          tunnel: w913 -> [w920 w922]
          frame False {
          }
          frame True {
            n223 = call "CONEX_FUNCTIONAL_GLOBAL.vi"("error in"=w922, "Command"=T22."CLOSE") -> ("error out"=w925:errorcluster)  [unwired: 7 in, 2 out]
            n224 = flat-sequence {
              tunnel: w925 -> [w928]
              tunnel: [w928] -> w924
              frame #0 {
                n225 = Wait (ms)(milliseconds to wait=u32 50) -> ()  [unwired: 1 out]
              }
            }
            n226 = local write "reset motor comm. link"(FALSE ("reset motor comm. link")) -> ()
            n227 = call "CONEX_FUNCTIONAL_GLOBAL.vi"("error in"=w924, "Command"=T22."INIT") -> ("error out"=w923:errorcluster)  [unwired: 7 in, 2 out]
          }
        }
        n228 = call "CONEX_FUNCTIONAL_GLOBAL.vi"("Axis"=enum16{"X", "Y", "Z", "XY", "XZ", "YZ", "XYZ"}."XYZ", "error in"=w914, "Command"=T22."GET POS") -> ("error out"=w912:errorcluster, "Current Position"=w916:dbl[])  [unwired: 6 in, 1 out]
        n229 = local write "Current Position"(w916) -> ()
      }
      frame True {
        # "put cursor somewhere\nwhere mouse clicks and \nmouse wheel moves won't\nbe heard by the window"
        n230 = Not(x=w938) -> (.not. x?=w939:bool)
        n231 = Quotient & Remainder(x=w933, y=10) -> (x-y*floor(x/y)=w931:i32)  [unwired: 1 out]
        n232 = case shown="True" w939 {
          tunnel: w937 -> [w964 w968]
          tunnel: [w964 w967] -> w936
          tunnel: w935 -> [w963 w966]
          tunnel: [w963 w965] -> w934
          frame False {
          }
          frame True {
            n233 = call-poly <vilib>:"Acquire Input Data.vi"("device ID"=w968, "error in (no error)"=w966) -> ("device ID"=w967:refnum<k1>, "error out"=w965:errorcluster)  [unwired: 14 in, 2 out]
          }
        }
        n234 = Equal To 0?(x=w931) -> (x = 0?=w930:bool)
        n235 = case shown="True" w930 {
          frame False {
          }
          frame True {
            # "SetCursorPos"
            n236 = dll-call lib="User32.dll" fn="SetCursorPos"(900, 600) -> ()  [unwired: 5 in, 3 out]
          }
        }
        n237 = call-poly <vilib>:"Acquire Input Data.vi"("device ID"=w936, "key mode"=enum16{"RELATIVE", "ABSOLUTE"}."RELATIVE", "error in (no error)"=w934) -> ("device ID"=w960:refnum<k1>, "axis info"=w958:T31, "error out"=w940:errorcluster)  [unwired: 13 in, 1 out]
        n238 = Cluster To Array(cluster=w958) -> (array=w956:i32[])
        n239 = Compound Arithmetic op=MULTIPLY(invert 10000.0 ("value"), "mouse sensitivity", w956) -> (w954:dbl[])
        n240 = call "subVI_explode3array.vi"("Array"=w954) -> ("x"=w945:dbl, "y"=w944:dbl, "z"=w953:dbl)  [unwired: 12 in]
        n241 = case shown="False" "invert y?" {
          tunnel: w944 -> [w969 w971]
          tunnel: [w969 w970] -> w943
          frame False {
          }
          frame True {
            n242 = Negate(x=w971) -> (-x=w970:dbl)
          }
        }
        n243 = case shown="False" "invert x?" {
          tunnel: w945 -> [w972 w974]
          tunnel: [w972 w973] -> w942
          frame False {
          }
          frame True {
            n244 = Negate(x=w974) -> (-x=w973:dbl)
          }
        }
        n245 = Divide(x=w953, y=50.0) -> (x/y=w951:dbl)
        n246 = Build Array(w942, w943, w951) -> (w948:dbl[])
        n247 = call "CONEX_FUNCTIONAL_GLOBAL.vi"("Axis"=enum16{"X", "Y", "Z", "XY", "XZ", "YZ", "XYZ"}."XYZ", "error in"=w940, "Position"=w948, "Command"=T22."REL MOVE") -> ("error out"=w941:errorcluster)  [unwired: 5 in, 2 out]
      }
    }
    n248 = local read "Stop All"() -> (w905:bool)
    n249 = node-c288() -> ()  [unwired: 1 in, 1 out]
  }
  n250 = node-c288(i64 1 ("Period"), 1 ("Processor")) -> (w163:T26)  [unwired: 2 out]
  n251 = node-c288(2 ("Processor")) -> (w7:T26)  [unwired: 3 in]
  n252 = node-c288() -> (w68:T26)  [unwired: 4 in]
  n253 = node-c288() -> (w75:T26)  [unwired: 4 out]
  n254 = timed-loop "Acquire Data" {
    tunnel: w16 -> [w1229]
    tunnel: w39 -> [w1228]
    tunnel: [w1259] -> w30
    tunnel: [w1253] -> w29
    timing: w163 -> [_]
    timing-out: [_] -> w162
    tunnel: w58 -> [w1057]
    stop <- "Stop All" stop-if-true
    (unwired) u32 0 ("Number of Elements")
    w1044 = "NI_ChannelName" ("name")
    n255 = node-c288() -> ()  [unwired: 2 out]
    n256 = First Call?() -> (First Call?: T/F=w1010:bool)
    n257 = Or(x="Reset", y=w1010) -> (x .or. y?=w1011:bool)
    n258 = case "Reset data stream" shown="True" w1011 {
      tunnel: w1229 -> [w1345 w1353]
      tunnel: w1228 -> [w1344 w1352]
      tunnel: [w1345 w1347] -> w1224
      tunnel: [w1344 w1346] -> w1223
      frame False {
      }
      frame True {
        w1350 = TRUE ("AI to FIFO")
        n259 = local write "Overflow (data lost)"(FALSE ("Overflow (data lost)")) -> ()
        n260 = call "reset FPGA DMA.vi"("error in"=w1352, "FPGA VI Reference In"=w1353) -> ("error out"=w1348:errorcluster, "FPGA VI Reference Out"=w1349:T19)
        n261 = xnode "Read/Write Control"("FPGA VI Reference In"=w1349, "error in"=w1348, "AI to FIFO"=w1350, "APD to FIFO"=w1350) -> ("FPGA VI Reference Out"=w1347:T19, "error out"=w1346:errorcluster)
      }
    }
    n262 = Or(x="Start AOD Scan", y="Trap Raster Scan") -> (x .or. y?=w1174:bool)
    n263 = case "Start AOM raster scan" shown="False" w1174 {
      tunnel: w1224 -> [w2953 w2963]
      tunnel: w1223 -> [w2952 w2962]
      tunnel: [w2953 w2956] -> w1222
      tunnel: [w2952 w2955] -> w1221
      frame False {
      }
      frame True {
        n264 = case shown="True" "Restart DMA? (AOD)" {
          tunnel: [w3374 w3376] -> w2957
          tunnel: [w3373 w3375] -> w2958
          tunnel: w2963 -> [w3374 w3378]
          tunnel: w2962 -> [w3373 w3377]
          frame False {
          }
          frame True {
            n265 = local write "Overflow (data lost)"(FALSE ("Overflow (data lost)")) -> ()
            n266 = call "reset FPGA DMA.vi"("error in"=w3377, "FPGA VI Reference In"=w3378) -> ("error out"=w3375:errorcluster, "FPGA VI Reference Out"=w3376:T19)
          }
        }
        n267 = local write "Trap Raster Scan"(FALSE ("Trap Raster Scan")) -> ()
        n268 = case shown="True" "Move MCL Also?" {
          tunnel: w2958 -> [w2966 w3075]
          tunnel: w2957 -> [w2967 w3076]
          tunnel: [w2965 w3079] -> w2956
          tunnel: [w2964 w3078] -> w2955
          frame False {
            w2968 = TRUE ("AI to FIFO")
            n269 = xnode "Read/Write Control"("FPGA VI Reference In"=w2967, "error in"=w2966, "AI to FIFO"=w2968, "APD to FIFO"=w2968, "Start scan"=w2968) -> ("FPGA VI Reference Out"=w2965:T19, "error out"=w2964:errorcluster)
          }
          frame True {
            w3072 = FALSE ("1D or 2D Scan?")
            w3077 = TRUE ("AI to FIFO")
            # "Count for MCL loop"
            # "N total cycles"
            # "N steps"
            # "V_int"
            n270 = local read "Scan Range (nm)"() -> (w3054:dbl)
            n271 = local read "Number of F/B Scans (AOD)"() -> (w3071:u16)
            n272 = Sign(1:w3054) -> (0:w3053:dbl)
            n273 = Compound Arithmetic op=MULTIPLY(w3054, "MCL Step Position Ratio", "MCL/AOM Scale Tweak") -> (w3058:dbl)
            n274 = Negate(x=w3053) -> (-x=w3050:dbl)
            n275 = Multiply(x=w3050, y="MCL Step Increment (V_int)") -> (x*y=w3052:dbl)
            n276 = Divide(x=w3058, y="MCL X Cal (nm/V)") -> (x/y=w3064:dbl)
            n277 = Multiply(x=32767.0 ("y"), y=w3064) -> (x*y=w3070:dbl)
            n278 = local read "Total Counts (ticks)"() -> (w3055:u32)
            n279 = local read "Cycles/step (AOD)"() -> (w3066:u64)
            n280 = local read "Scan steps (AOD)"() -> (w3067:u64)
            n281 = Divide(x=w3070, y=10.0) -> (x/y=w3063:dbl)
            n282 = Divide(x=w3063, y="MCL Step Increment (V_int)") -> (x/y=w3061:dbl)
            n283 = Absolute Value(x=w3061) -> (abs(x)=w3049:dbl)
            n284 = Compound Arithmetic op=MULTIPLY(w3067, w3066, w3055) -> (w3062:u64)
            n285 = local write "wait to reset values"(w3077) -> ()
            n286 = local write "MCL Scanning"(w3077) -> ()
            n287 = Divide(x=w3062, y=w3049) -> (x/y=w3059:dbl)
            "MCL Count" <- w3059
            n288 = xnode "Read/Write Control"("FPGA VI Reference In"=w3076, "error in"=w3075, "Scan steps (MCL)"=w3049, "Number of scans (MCL)"=w3071, "Cycles per step (MCL)"=u64 1, "Scan freq.  increment (MCL)"=w3052, "1D or 2D Scan?"=w3072, "MCL Scan Axis"=w3072, "Cont. Scan (MCL)"=w3072, "MCL count"=w3059) -> ("FPGA VI Reference Out"=w3074:T19, "error out"=w3073:errorcluster)
            n289 = xnode "Read/Write Control"("FPGA VI Reference In"=w3074, "error in"=w3073, "AI to FIFO"=w3077, "APD to FIFO"=w3077, "Start scan"=w3077, "Start scan (MCL)"=w3077) -> ("FPGA VI Reference Out"=w3079:T19, "error out"=w3078:errorcluster)